vi "Dresden R2R Sputter 03.02.2018 IY24.vi"() -> ()   [LabVIEW 2009] (continued)
          tunnel: w9769 -> [w9795 w9871 w9895 w9919 w9956 w9990 w10014]
          tunnel: w9772 -> [w9794 w9870 w9894 w9918 w9955 w9989 w10013]
          frame #0 {
            n6486 = stacked-sequence {
              tunnel: [_ _ _ w9837 _] -> w9797
              tunnel: [_ _ _ w9828 _] -> w9796
              tunnel: w9795 -> [_ w9800 _ _ _]
              tunnel: w9794 -> [_ w9799 _ _ _]
              frame #0 {
                n6487 = Wait (ms)(milliseconds to wait=i32? 50) -> ()  [unwired: 1 out]
              }
              frame #1 {
                n6488 = Concatenate Strings("#003A:" ("string"), "\n", "\n") -> (w9818)
                n6489 = VISA Write(VISA resource name=w9800, write buffer=w9818, error in (no error)=w9799) -> (VISA resource name out=w9816, error out=w9815)  [unwired: 1 out]
                n6490 = stacked-sequence {
                  tunnel: [w9823] -> w9814
                  tunnel: w9816 -> [w9823]
                  tunnel: [w9822] -> w9813
                  tunnel: w9815 -> [w9822]
                  frame #0 {
                    n6491 = Wait (ms)(milliseconds to wait=i32? 50) -> ()  [unwired: 1 out]
                  }
                }
                n6492 = property class="Instr"(reference=w9814, error in=w9813) -> (reference out=w9810, error out=w9812, "Serial Settings:Number of Bytes at Serial Port"=w9811)
                n6493 = VISA Read(VISA resource name=w9810, byte count=w9811, error in (no error)=w9812) -> (VISA resource name out=w9802, read buffer=w9804, error out=w9801)  [unwired: 1 out]
                "read buffer 6" <- w9804
                n6494 = Match Pattern(string=w9804, regular expression="#003A:") -> (after substring=w9808)  [unwired: 1 in, 3 out]
                n6495 = String Subset(string=w9808, offset (0)=data[5B], length (rest)=i32? 3 ("length (rest)")) -> (substring=w9805)
                n6496 = Decimal String To Number(string=w9805) -> (number=→"Pc_bv3_position")  [unwired: 2 in, 1 out]
              }
              frame #2 {
                n6497 = Wait (ms)(milliseconds to wait=i32? 50) -> ()  [unwired: 1 out]
              }
              frame #3 {
                n6498 = Concatenate Strings("#003P:" ("string"), "\n", "\n") -> (w9851)
                n6499 = VISA Write(VISA resource name=w9836, write buffer=w9851, error in (no error)=w9835) -> (VISA resource name out=w9849, error out=w9848)  [unwired: 1 out]
                n6500 = stacked-sequence {
                  tunnel: [w9857] -> w9847
                  tunnel: w9849 -> [w9857]
                  tunnel: [w9856] -> w9846
                  tunnel: w9848 -> [w9856]
                  frame #0 {
                    n6501 = Wait (ms)(milliseconds to wait=i32? 50) -> ()  [unwired: 1 out]
                  }
                }
                n6502 = property class="Instr"(reference=w9847, error in=w9846) -> (reference out=w9843, error out=w9845, "Serial Settings:Number of Bytes at Serial Port"=w9844)
                n6503 = VISA Read(VISA resource name=w9843, byte count=w9844, error in (no error)=w9845) -> (VISA resource name out=w9837, read buffer=w9838, error out=w9828)  [unwired: 1 out]
                "read buffer 7" <- w9838
                n6504 = Match Pattern(string=w9838, regular expression="#003P:") -> (after substring=w9829)  [unwired: 1 in, 3 out]
                n6505 = String Subset(string=w9829, offset (0)=i32? 2, length (rest)=i32? 4 ("length (rest)")) -> (substring=w9839)
                n6506 = String Subset(string=w9829, offset (0)=data[5B], length (rest)=i32? 1 ("length (rest)")) -> (substring=w9827)
                n6507 = Equal?(x=w9827, y="-" ("substring")) -> (x = y?=w9825)
                n6508 = Decimal String To Number(string=w9839) -> (number=w9834)  [unwired: 2 in, 1 out]
                n6509 = case shown="True" w9825 {
                  frame #0 {
                  }
                  frame #1 {
                    w9854 = data[5B] ("Pressure_ch3")
                    n6510 = local write "Pressure_ch3"(w9854) -> ()
                    n6511 = local write "Pressure ch3_gui"(w9854) -> ()
                    n6512 = local write "Pressure ch3_gui2"(w9854) -> ()
                  }
                }
                n6513 = Divide(x=w9834, y=i32? 100) -> (x/y=→"Pressure_ch3" →"Pressure ch3_gui" →"Pressure ch3_gui2")
              }
              frame #4 {
                n6514 = Wait (ms)(milliseconds to wait=i32? 50) -> ()  [unwired: 1 out]
              }
            }
          }
          frame #1 {
            n6515 = Concatenate Strings("#003O:" ("string"), "\n", "\n") -> (w9874)
            n6516 = VISA Write(VISA resource name=w9871, write buffer=w9874, error in (no error)=w9870) -> (VISA resource name out=w9860, error out=w9862)  [unwired: 1 out]
            n6517 = stacked-sequence {
              tunnel: [w9882] -> w9869
              tunnel: w9860 -> [w9882]
              tunnel: [w9881] -> w9868
              tunnel: w9862 -> [w9881]
              frame #0 {
                n6518 = Wait (ms)(milliseconds to wait=i32? 50) -> ()  [unwired: 1 out]
              }
            }
            n6519 = property class="Instr"(reference=w9869, error in=w9868) -> (reference out=w9865, error out=w9867, "Serial Settings:Number of Bytes at Serial Port"=w9866)
            n6520 = local write "Pc_bv3_auto_open"(i16? 0 ("Pc_bv3_auto_open")) -> ()
            n6521 = VISA Read(VISA resource name=w9865, byte count=w9866, error in (no error)=w9867) -> (VISA resource name out=w9864, error out=w9863)  [unwired: 2 out]
            n6522 = stacked-sequence {
              tunnel: [w9879] -> w9859
              tunnel: w9864 -> [w9879]
              tunnel: [w9878] -> w9861
              tunnel: w9863 -> [w9878]
              frame #0 {
                n6523 = Wait (ms)(milliseconds to wait=i32? 50) -> ()  [unwired: 1 out]
              }
            }
          }
          frame #2 {
            n6524 = Concatenate Strings("#003C:" ("string"), "\n", "\n") -> (w9898)
            n6525 = VISA Write(VISA resource name=w9895, write buffer=w9898, error in (no error)=w9894) -> (VISA resource name out=w9886, error out=w9885)  [unwired: 1 out]
            n6526 = stacked-sequence {
              tunnel: [w9906] -> w9893
              tunnel: w9886 -> [w9906]
              tunnel: [w9905] -> w9892
              tunnel: w9885 -> [w9905]
              frame #0 {
                n6527 = Wait (ms)(milliseconds to wait=i32? 50) -> ()  [unwired: 1 out]
              }
            }
            n6528 = local write "Pc_bv3_auto_close"(i16? 0 ("Pc_bv3_auto_close")) -> ()
            n6529 = property class="Instr"(reference=w9893, error in=w9892) -> (reference out=w9889, error out=w9891, "Serial Settings:Number of Bytes at Serial Port"=w9890)
            n6530 = VISA Read(VISA resource name=w9889, byte count=w9890, error in (no error)=w9891) -> (VISA resource name out=w9888, error out=w9887)  [unwired: 2 out]
            n6531 = stacked-sequence {
              tunnel: [w9903] -> w9884
              tunnel: w9888 -> [w9903]
              tunnel: [w9902] -> w9883
              tunnel: w9887 -> [w9902]
              frame #0 {
                n6532 = Wait (ms)(milliseconds to wait=i32? 50) -> ()  [unwired: 1 out]
              }
            }
          }
          frame #3 {
            n6533 = In Range and Coerce(upper limit=dbl? 100.0, x="Set_position_value 3", lower limit=data[9B]) -> (coerced(x)=w9924)  [unwired: 1 out]
            n6534 = Multiply(x=w9924, y=dbl? 1000.0) -> (x*y=w9928)
            n6535 = Number To Decimal String(number=w9928) -> (decimal integer string=w9930)  [unwired: 1 out]
            n6536 = Concatenate Strings("000000" ("string"), w9930) -> (w9932)
            n6537 = String Length(string=w9932) -> (length=w9933)
            n6538 = Subtract(x=w9933, y=i32? 6) -> (x-y=w9935)
            n6539 = String Subset(string=w9932, offset (0)=w9935) -> (substring=w9925)  [unwired: 1 out]
            n6540 = Concatenate Strings("#003R:" ("string"), w9925, "\n", "\n") -> (w9937)
            n6541 = VISA Write(VISA resource name=w9919, write buffer=w9937, error in (no error)=w9918) -> (VISA resource name out=w9912, error out=w9910)  [unwired: 1 out]
            n6542 = stacked-sequence {
              tunnel: [w9942] -> w9911
              tunnel: w9912 -> [w9942]
              tunnel: w9910 -> [w9941]
              tunnel: [w9941] -> w9909
              frame #0 {
                n6543 = Wait (ms)(milliseconds to wait=i32? 50) -> ()  [unwired: 1 out]
              }
            }
            n6544 = property class="Instr"(reference=w9911, error in=w9909) -> (reference out=w9915, error out=w9917, "Serial Settings:Number of Bytes at Serial Port"=w9916)
            n6545 = VISA Read(VISA resource name=w9915, byte count=w9916, error in (no error)=w9917) -> (VISA resource name out=w9914, error out=w9913)  [unwired: 2 out]
            n6546 = local write "Pc_bv3_auto_set position"(i16? 0 ("Pc_bv3_auto_set position")) -> ()
            n6547 = stacked-sequence {
              tunnel: [w9940] -> w9908
              tunnel: w9914 -> [w9940]
              tunnel: [w9939] -> w9907
              tunnel: w9913 -> [w9939]
              frame #0 {
                n6548 = Wait (ms)(milliseconds to wait=i32? 50) -> ()  [unwired: 1 out]
              }
            }
          }
          frame #4 {
            n6549 = Multiply(x="Set_pressure_value 3", y=dbl? 10000.0) -> (x*y=w9962)
            n6550 = Number To Decimal String(number=w9962) -> (decimal integer string=w9964)  [unwired: 1 out]
            n6551 = Concatenate Strings("00000000" ("string"), w9964) -> (w9966)
            n6552 = String Length(string=w9966) -> (length=w9967)
            n6553 = Subtract(x=w9967, y=i32? 8) -> (x-y=w9969)
            n6554 = String Subset(string=w9966, offset (0)=w9969) -> (substring=w9959)  [unwired: 1 out]
            n6555 = Concatenate Strings("#003S:" ("string"), w9959, "\n", "\n") -> (w9971)
            n6556 = VISA Write(VISA resource name=w9956, write buffer=w9971, error in (no error)=w9955) -> (VISA resource name out=w9948, error out=w9946)  [unwired: 1 out]
            n6557 = stacked-sequence {
              tunnel: [w9976] -> w9949
              tunnel: w9948 -> [w9976]
              tunnel: [w9975] -> w9947
              tunnel: w9946 -> [w9975]
              frame #0 {
                n6558 = Wait (ms)(milliseconds to wait=i32? 50) -> ()  [unwired: 1 out]
              }
            }
            n6559 = property class="Instr"(reference=w9949, error in=w9947) -> (reference out=w9952, error out=w9954, "Serial Settings:Number of Bytes at Serial Port"=w9953)
            n6560 = local write "Pc_bv3_auto_set_pressure"(i16? 0 ("Pc_bv3_auto_set_pressure")) -> ()
            n6561 = VISA Read(VISA resource name=w9952, byte count=w9953, error in (no error)=w9954) -> (VISA resource name out=w9951, error out=w9950)  [unwired: 2 out]
            n6562 = stacked-sequence {
              tunnel: [w9974] -> w9945
              tunnel: w9951 -> [w9974]
              tunnel: [w9973] -> w9944
              tunnel: w9950 -> [w9973]
              frame #0 {
                n6563 = Wait (ms)(milliseconds to wait=i32? 50) -> ()  [unwired: 1 out]
              }
            }
          }
          frame #5 {
            n6564 = Concatenate Strings("#003Z:" ("string"), "\n", "\n") -> (w9993)
            n6565 = VISA Write(VISA resource name=w9990, write buffer=w9993, error in (no error)=w9989) -> (VISA resource name out=w9982, error out=w9980)  [unwired: 1 out]
            n6566 = stacked-sequence {
              tunnel: [w10000] -> w9983
              tunnel: w9982 -> [w10000]
              tunnel: [w9999] -> w9981
              tunnel: w9980 -> [w9999]
              frame #0 {
                n6567 = Wait (ms)(milliseconds to wait=i32? 50) -> ()  [unwired: 1 out]
              }
            }
            n6568 = local write "Pc_bv3_auto_baratron_set_zero"(i16? 0 ("Pc_bv3_auto_baratron_set_zero")) -> ()
            n6569 = property class="Instr"(reference=w9983, error in=w9981) -> (reference out=w9986, error out=w9988, "Serial Settings:Number of Bytes at Serial Port"=w9987)
            n6570 = VISA Read(VISA resource name=w9986, byte count=w9987, error in (no error)=w9988) -> (VISA resource name out=w9985, error out=w9984)  [unwired: 2 out]
            n6571 = stacked-sequence {
              tunnel: [w9998] -> w9979
              tunnel: w9985 -> [w9998]
              tunnel: [w9997] -> w9978
              tunnel: w9984 -> [w9997]
              frame #0 {
                n6572 = Wait (ms)(milliseconds to wait=i32? 50) -> ()  [unwired: 1 out]
              }
            }
          }
          frame #6 {
            n6573 = Concatenate Strings("#003s:" ("string"), "string", "\n", "\n") -> (w10019)
            n6574 = VISA Write(VISA resource name=w10014, write buffer=w10019, error in (no error)=w10013) -> (VISA resource name out=w10006, error out=w10004)  [unwired: 1 out]
            n6575 = stacked-sequence {
              tunnel: [w10024] -> w10007
              tunnel: w10006 -> [w10024]
              tunnel: [w10023] -> w10005
              tunnel: w10004 -> [w10023]
              frame #0 {
                n6576 = Wait (ms)(milliseconds to wait=i32? 50) -> ()  [unwired: 1 out]
              }
            }
            n6577 = property class="Instr"(reference=w10007, error in=w10005) -> (reference out=w10010, error out=w10012, "Serial Settings:Number of Bytes at Serial Port"=w10011)
            n6578 = VISA Read(VISA resource name=w10010, byte count=w10011, error in (no error)=w10012) -> (VISA resource name out=w10009, error out=w10008)  [unwired: 2 out]
            n6579 = stacked-sequence {
              tunnel: [w10022] -> w10003
              tunnel: w10009 -> [w10022]
              tunnel: [w10021] -> w10002
              tunnel: w10008 -> [w10021]
              frame #0 {
                n6580 = Wait (ms)(milliseconds to wait=i32? 50) -> ()  [unwired: 1 out]
              }
            }
          }
        }
      }
      frame #3 {
        n6581 = Compound Arithmetic op=OR("Pc_bv4_open", "Pc_bv_open_ch4_gui", "Pc_bv4_auto_open", "Pc_bv4_open 2") -> (w10032)
        n6582 = Or(x="Pc_bv4_set position", y="Pc_bv4_auto_set position") -> (x .or. y?=w10043)
        n6583 = Or(x="Pc_bv4_set_pressure", y="Pc_bv4_auto_set_pressure") -> (x .or. y?=w10042)
        n6584 = Or(x="Pc_bv4_auto_baratron_set_zero", y="Baratron_set_zero") -> (x .or. y?=w10041)
        n6585 = Compound Arithmetic op=OR("Pc_bv4_close", "Pc_bv_close_ch4_gui", "Pc_bv4_auto_close", "Pc_bv4_close 2") -> (w10033)
        n6586 = Build Array(i16? 0, w10032, w10033, w10043, w10042, w10041) -> (w10040)
        n6587 = Boolean Array To Number(Boolean array=w10040) -> (number=w10052)
        n6588 = Mantissa & Exponent(0:w10052) -> (2:w10051)  [unwired: 1 out]
        n6589 = case shown="3" w10051 {
          tunnel: [w10056 w10119 w10143 w10166 w10205 w10238] -> w10031
          tunnel: [w10055 w10118 w10142 w10167 w10204 w10237] -> w10030
          tunnel: w10029 -> [w10054 w10130 w10154 w10178 w10216 w10249]
          tunnel: w10028 -> [w10053 w10129 w10153 w10177 w10215 w10248]
          frame #0 {
            n6590 = stacked-sequence {
              tunnel: [_ _ _ w10096 _] -> w10056
              tunnel: [_ _ _ w10095 _] -> w10055
              tunnel: w10054 -> [_ w10059 _ _ _]
              tunnel: w10053 -> [_ w10058 _ _ _]
              frame #0 {
                n6591 = Wait (ms)(milliseconds to wait=i32? 50) -> ()  [unwired: 1 out]
              }
              frame #1 {
                n6592 = Concatenate Strings("#004A:" ("string"), "\n", "\n") -> (w10077)
                n6593 = VISA Write(VISA resource name=w10059, write buffer=w10077, error in (no error)=w10058) -> (VISA resource name out=w10075, error out=w10074)  [unwired: 1 out]
                n6594 = stacked-sequence {
                  tunnel: [w10082] -> w10073
                  tunnel: w10075 -> [w10082]
                  tunnel: [w10081] -> w10072
                  tunnel: w10074 -> [w10081]
                  frame #0 {
                    n6595 = Wait (ms)(milliseconds to wait=i32? 50) -> ()  [unwired: 1 out]
                  }
                }
                n6596 = property class="Instr"(reference=w10073, error in=w10072) -> (reference out=w10069, error out=w10071, "Serial Settings:Number of Bytes at Serial Port"=w10070)
                n6597 = VISA Read(VISA resource name=w10069, byte count=w10070, error in (no error)=w10071) -> (VISA resource name out=w10061, read buffer=w10063, error out=w10060)  [unwired: 1 out]
                "read buffer 8" <- w10063
                n6598 = Match Pattern(string=w10063, regular expression="#004A:") -> (after substring=w10067)  [unwired: 1 in, 3 out]
                n6599 = String Subset(string=w10067, offset (0)=data[5B], length (rest)=i32? 3 ("length (rest)")) -> (substring=w10064)
                n6600 = Decimal String To Number(string=w10064) -> (number=→"Pc_bv4_position")  [unwired: 2 in, 1 out]
              }
              frame #2 {
                n6601 = Wait (ms)(milliseconds to wait=i32? 50) -> ()  [unwired: 1 out]
              }
              frame #3 {
                n6602 = Concatenate Strings("#004P:" ("string"), "\n", "\n") -> (w10110)
                n6603 = VISA Write(VISA resource name=w10094, write buffer=w10110, error in (no error)=w10090) -> (VISA resource name out=w10108, error out=w10107)  [unwired: 1 out]
                n6604 = stacked-sequence {
                  tunnel: [w10116] -> w10106
                  tunnel: w10108 -> [w10116]
                  tunnel: [w10115] -> w10105
                  tunnel: w10107 -> [w10115]
                  frame #0 {
                    n6605 = Wait (ms)(milliseconds to wait=i32? 50) -> ()  [unwired: 1 out]
                  }
                }
                n6606 = property class="Instr"(reference=w10106, error in=w10105) -> (reference out=w10102, error out=w10104, "Serial Settings:Number of Bytes at Serial Port"=w10103)
                n6607 = VISA Read(VISA resource name=w10102, byte count=w10103, error in (no error)=w10104) -> (VISA resource name out=w10096, read buffer=w10097, error out=w10095)  [unwired: 1 out]
                "read buffer 9" <- w10097
                n6608 = Match Pattern(string=w10097, regular expression="#004P:") -> (after substring=w10084)  [unwired: 1 in, 3 out]
                n6609 = String Subset(string=w10084, offset (0)=data[5B], length (rest)=i32? 1 ("length (rest)")) -> (substring=w10087)
                n6610 = String Subset(string=w10084, offset (0)=i32? 2, length (rest)=i32? 4 ("length (rest)")) -> (substring=w10098)
                n6611 = Equal?(x=w10087, y="-") -> (x = y?=w10085)
                n6612 = Decimal String To Number(string=w10098) -> (number=w10093)  [unwired: 2 in, 1 out]
                n6613 = case shown="True" w10085 {
                  frame #0 {
                  }
                  frame #1 {
                    w10113 = data[5B] ("Pressure 4")
                    n6614 = local write "Pressure 4"(w10113) -> ()
                    n6615 = local write "Pressurech4_gui"(w10113) -> ()
                    n6616 = local write "Pressurech4_gui 2"(w10113) -> ()
                  }
                }
                n6617 = Divide(x=w10093, y=i32? 100) -> (x/y=→"Pressure 4" →"Pressurech4_gui" →"Pressurech4_gui 2")
              }
              frame #4 {
                n6618 = Wait (ms)(milliseconds to wait=i32? 50) -> ()  [unwired: 1 out]
              }
            }
          }
          frame #1 {
            n6619 = Concatenate Strings("#004O:" ("string"), "\n", "\n") -> (w10133)
            n6620 = VISA Write(VISA resource name=w10130, write buffer=w10133, error in (no error)=w10129) -> (VISA resource name out=w10122, error out=w10120)  [unwired: 1 out]
            n6621 = stacked-sequence {
              tunnel: [w10140] -> w10123
              tunnel: w10122 -> [w10140]
              tunnel: [w10139] -> w10121
              tunnel: w10120 -> [w10139]
              frame #0 {
                n6622 = Wait (ms)(milliseconds to wait=i32? 50) -> ()  [unwired: 1 out]
              }
            }
            n6623 = local write "Pc_bv4_auto_open"(i16? 0 ("Pc_bv4_auto_open")) -> ()
            n6624 = property class="Instr"(reference=w10123, error in=w10121) -> (reference out=w10126, error out=w10128, "Serial Settings:Number of Bytes at Serial Port"=w10127)
            n6625 = VISA Read(VISA resource name=w10126, byte count=w10127, error in (no error)=w10128) -> (VISA resource name out=w10125, error out=w10124)  [unwired: 2 out]
            n6626 = stacked-sequence {
              tunnel: [w10138] -> w10119
              tunnel: w10125 -> [w10138]
              tunnel: [w10137] -> w10118
              tunnel: w10124 -> [w10137]
              frame #0 {
                n6627 = Wait (ms)(milliseconds to wait=i32? 50) -> ()  [unwired: 1 out]
              }
            }
          }
          frame #2 {
            n6628 = Concatenate Strings("#004C:" ("string"), "\n", "\n") -> (w10157)
            n6629 = VISA Write(VISA resource name=w10154, write buffer=w10157, error in (no error)=w10153) -> (VISA resource name out=w10145, error out=w10144)  [unwired: 1 out]
            n6630 = local write "Pc_bv4_auto_close"(i16? 0 ("Pc_bv4_auto_close")) -> ()
            n6631 = stacked-sequence {
              tunnel: [w10164] -> w10147
              tunnel: w10145 -> [w10164]
              tunnel: [w10163] -> w10146
              tunnel: w10144 -> [w10163]
              frame #0 {
                n6632 = Wait (ms)(milliseconds to wait=i32? 50) -> ()  [unwired: 1 out]
              }
            }
            n6633 = property class="Instr"(reference=w10147, error in=w10146) -> (reference out=w10150, error out=w10152, "Serial Settings:Number of Bytes at Serial Port"=w10151)
            n6634 = VISA Read(VISA resource name=w10150, byte count=w10151, error in (no error)=w10152) -> (VISA resource name out=w10149, error out=w10148)  [unwired: 2 out]
            n6635 = stacked-sequence {
              tunnel: [w10162] -> w10143
              tunnel: w10149 -> [w10162]
              tunnel: [w10161] -> w10142
              tunnel: w10148 -> [w10161]
              frame #0 {
                n6636 = Wait (ms)(milliseconds to wait=i32? 50) -> ()  [unwired: 1 out]
              }
            }
          }
          frame #3 {
            n6637 = In Range and Coerce(upper limit=dbl? 100.0, x="Set_position_value 4", lower limit=data[9B]) -> (coerced(x)=w10181)  [unwired: 1 out]
            n6638 = Multiply(x=w10181, y=dbl? 1000.0) -> (x*y=w10188)
            n6639 = Number To Decimal String(number=w10188) -> (decimal integer string=w10189)  [unwired: 1 out]
            n6640 = Concatenate Strings("000000" ("string"), w10189) -> (w10191)
            n6641 = String Length(string=w10191) -> (length=w10192)
            n6642 = Subtract(x=w10192, y=i32? 6) -> (x-y=w10194)
            n6643 = String Subset(string=w10191, offset (0)=w10194) -> (substring=w10185)  [unwired: 1 out]
            n6644 = Concatenate Strings("#004R:" ("string"), w10185, "\n", "\n") -> (w10196)
            n6645 = VISA Write(VISA resource name=w10178, write buffer=w10196, error in (no error)=w10177) -> (VISA resource name out=w10169, error out=w10168)  [unwired: 1 out]
            n6646 = stacked-sequence {
              tunnel: [w10201] -> w10171
              tunnel: w10169 -> [w10201]
              tunnel: [w10200] -> w10170
              tunnel: w10168 -> [w10200]
              frame #0 {
                n6647 = Wait (ms)(milliseconds to wait=i32? 50) -> ()  [unwired: 1 out]
              }
            }
            n6648 = property class="Instr"(reference=w10171, error in=w10170) -> (reference out=w10174, error out=w10176, "Serial Settings:Number of Bytes at Serial Port"=w10175)
            n6649 = local write "Pc_bv4_auto_set position"(i16? 0 ("Pc_bv4_auto_set position")) -> ()
            n6650 = VISA Read(VISA resource name=w10174, byte count=w10175, error in (no error)=w10176) -> (VISA resource name out=w10173, error out=w10172)  [unwired: 2 out]
            n6651 = stacked-sequence {
              tunnel: [w10199] -> w10166
              tunnel: w10173 -> [w10199]
              tunnel: [w10198] -> w10167
              tunnel: w10172 -> [w10198]
              frame #0 {
                n6652 = Wait (ms)(milliseconds to wait=i32? 50) -> ()  [unwired: 1 out]
              }
            }
          }
          frame #4 {
            n6653 = Multiply(x="Set_pressure_value 4", y=dbl? 10000.0) -> (x*y=w10221)
            n6654 = Number To Decimal String(number=w10221) -> (decimal integer string=w10223)  [unwired: 1 out]
            n6655 = Concatenate Strings("00000000" ("string"), w10223) -> (w10225)
            n6656 = String Length(string=w10225) -> (length=w10226)
            n6657 = Subtract(x=w10226, y=i32? 8) -> (x-y=w10228)
            n6658 = String Subset(string=w10225, offset (0)=w10228) -> (substring=w10218)  [unwired: 1 out]
            n6659 = Concatenate Strings("#004S:" ("string"), w10218, "\n", "\n") -> (w10230)
            n6660 = VISA Write(VISA resource name=w10216, write buffer=w10230, error in (no error)=w10215) -> (VISA resource name out=w10207, error out=w10206)  [unwired: 1 out]
            n6661 = stacked-sequence {
              tunnel: [w10235] -> w10209
              tunnel: w10207 -> [w10235]
              tunnel: [w10234] -> w10208
              tunnel: w10206 -> [w10234]
              frame #0 {
                n6662 = Wait (ms)(milliseconds to wait=i32? 50) -> ()  [unwired: 1 out]
              }
            }
            n6663 = property class="Instr"(reference=w10209, error in=w10208) -> (reference out=w10212, error out=w10214, "Serial Settings:Number of Bytes at Serial Port"=w10213)
            n6664 = local write "Pc_bv4_auto_set_pressure"(i16? 0 ("Pc_bv4_auto_set_pressure")) -> ()
            n6665 = VISA Read(VISA resource name=w10212, byte count=w10213, error in (no error)=w10214) -> (VISA resource name out=w10211, error out=w10210)  [unwired: 2 out]
            n6666 = stacked-sequence {
              tunnel: [w10233] -> w10205
              tunnel: w10211 -> [w10233]
              tunnel: [w10232] -> w10204
              tunnel: w10210 -> [w10232]
              frame #0 {
                n6667 = Wait (ms)(milliseconds to wait=i32? 50) -> ()  [unwired: 1 out]
              }
            }
          }
          frame #5 {
            n6668 = Concatenate Strings("#004Z:" ("string"), "\n", "\n") -> (w10252)
            n6669 = VISA Write(VISA resource name=w10249, write buffer=w10252, error in (no error)=w10248) -> (VISA resource name out=w10239, error out=w10240)  [unwired: 1 out]
            n6670 = stacked-sequence {
              tunnel: [w10259] -> w10242
              tunnel: w10239 -> [w10259]
              tunnel: [w10258] -> w10241
              tunnel: w10240 -> [w10258]
              frame #0 {
                n6671 = Wait (ms)(milliseconds to wait=i32? 50) -> ()  [unwired: 1 out]
              }
            }
            n6672 = local write "Pc_bv4_auto_baratron_set_zero"(i16? 0 ("Pc_bv4_auto_baratron_set_zero")) -> ()
            n6673 = property class="Instr"(reference=w10242, error in=w10241) -> (reference out=w10245, error out=w10247, "Serial Settings:Number of Bytes at Serial Port"=w10246)
            n6674 = VISA Read(VISA resource name=w10245, byte count=w10246, error in (no error)=w10247) -> (VISA resource name out=w10244, error out=w10243)  [unwired: 2 out]
            n6675 = stacked-sequence {
              tunnel: [w10257] -> w10238
              tunnel: w10244 -> [w10257]
              tunnel: [w10256] -> w10237
              tunnel: w10243 -> [w10256]
              frame #0 {
                n6676 = Wait (ms)(milliseconds to wait=i32? 50) -> ()  [unwired: 1 out]
              }
            }
          }
        }
      }
    }
    n6677 = Wait Until Next ms Multiple(millisecond multiple=i32? 300) -> ()  [unwired: 1 out]
  }
  n6678 = while {
    tunnel: w833 -> [w10265]
    tunnel: w832 -> [w10264]
    tunnel: [w10263] -> w811
    tunnel: [w10262] -> w810
    i -> [w10261]
    stop <- i16? 0 stop-if-true
    n6679 = Wait Until Next ms Multiple(millisecond multiple=i32? 300) -> ()  [unwired: 1 out]
    n6680 = stacked-sequence {
      tunnel: w10265 -> [w10320]
      tunnel: w10264 -> [w10298]
      tunnel: [w10297] -> w10263
      tunnel: [w10296] -> w10262
      tunnel: w10261 -> [w10304]
      frame #0 {
        n6681 = Compound Arithmetic op=OR("Dc_off", "Dc_auto_off", "Dc_off 2") -> (w10291)
        n6682 = Compound Arithmetic op=OR("Dc_host_auto", "DC_host", "DC_host 2") -> (w10268)
        n6683 = Compound Arithmetic op=OR("Dc_set", "Dc_set 2", "Dc_auto_set") -> (w10287)
        n6684 = Compound Arithmetic op=OR("Dc_auto_set_zero", "Dc_set_zero", "Dc_set_zero 2") -> (w10288)
        n6685 = Boolean To (0,1)(Boolean=w10291) -> (0, 1=w10300)
        n6686 = Boolean To (0,1)(Boolean=w10268) -> (0, 1=w10299)
        n6687 = Compound Arithmetic op=OR("Dc_auto_off_ramp_up", "DC_ramp_up", "DC_ramp_up 2") -> (w10289)
        n6688 = Compound Arithmetic op=OR("Dc_auto_ramp_down", "DC_ramp_down", "DC_ramp_down 2") -> (w10290)
        n6689 = Compound Arithmetic op=OR("Dc_on", "Dc_auto_on", "Dc_on 2") -> (w10292)
        n6690 = Boolean To (0,1)(Boolean=w10288) -> (0, 1=w10324)
        n6691 = Boolean To (0,1)(Boolean=w10287) -> (0, 1=w10328)
        n6692 = Multiply(x=w10299, y=i16? 1) -> (x*y=w10321)
        n6693 = Boolean To (0,1)(Boolean="DC_auto_voltage_mode") -> (0, 1=w10308)
        n6694 = Boolean To (0,1)(Boolean=w10289) -> (0, 1=w10318)
        n6695 = Boolean To (0,1)(Boolean=w10290) -> (0, 1=w10315)
        n6696 = Boolean To (0,1)(Boolean="DC_auto_power_mode") -> (0, 1=w10312)
        n6697 = Multiply(x=w10300, y=i16? 3) -> (x*y=w10329)
        n6698 = Multiply(x=w10324, y=i16? 5) -> (x*y=w10323)
        n6699 = Multiply(x=w10328, y=i16? 4) -> (x*y=w10326)
        n6700 = Multiply(x=w10308, y=i16? 9) -> (x*y=w10307)
        n6701 = Multiply(x=w10318, y=i16? 6) -> (x*y=w10314)
        n6702 = Multiply(x=w10315, y=i16? 7) -> (x*y=w10313)
        n6703 = Multiply(x=w10312, y=i16? 8) -> (x*y=w10310)
        n6704 = Boolean To (0,1)(Boolean=w10292) -> (0, 1=w10333)
        n6705 = Multiply(x=w10333, y=i16? 2) -> (x*y=w10331)
        n6706 = Compound Arithmetic op=ADD(w10321, w10331, w10329, w10326, w10323, w10314, w10313, w10310, w10307) -> (w10319)
        n6707 = Quotient & Remainder(x=w10304, y=i32? 5) -> (x-y*floor(x/y)=w10302)  [unwired: 1 out]
        n6708 = Equal To 0?(x=w10302) -> (x = 0?=w10301)
        n6709 = case shown="0, Default" w10319 {
          tunnel: w10320 -> [w10338 w10421 w10428 w10436 w10450 w10474 w10501 w10528 w10551 w10558]
          tunnel: w10298 -> [w10337 w10420 w10427 w10435 w10449 w10473 w10500 w10527 w10550 w10557]
          tunnel: [w10335 w10419 w10425 w10434 w10445 w10472 w10499 w10526 w10549 w10556] -> w10297
          tunnel: [w10334 w10418 w10424 w10433 w10444 w10471 w10498 w10525 w10548 w10555] -> w10296
          tunnel: w10301 -> [w10336 _ _ _ _ _ _ _ _ _]
          frame #0 {
            n6710 = case shown="True" w10336 {
              tunnel: w10338 -> [w10342 w10388]
              tunnel: w10337 -> [w10341 w10387]
              tunnel: [w10340 w10384] -> w10335
              tunnel: [w10339 w10385] -> w10334
              frame #0 {
                n6711 = VISA Write(VISA resource name=w10342, write buffer=bytes[3], error in (no error)=w10341) -> (VISA resource name out=w10365, error out=w10366)  [unwired: 1 out]
                n6712 = stacked-sequence {
                  tunnel: [w10382] -> w10363
                  tunnel: w10365 -> [w10382]
                  tunnel: [w10381] -> w10362
                  tunnel: w10366 -> [w10381]
                  frame #0 {
                    n6713 = Wait Until Next ms Multiple(millisecond multiple=i32? 40) -> ()  [unwired: 1 out]
                  }
                }
                n6714 = property class="Instr"(reference=w10363, error in=w10362) -> (reference out=w10357, error out=w10359, "Serial Settings:Number of Bytes at Serial Port"=w10358)
                n6715 = VISA Read(VISA resource name=w10357, byte count=w10358, error in (no error)=w10359) -> (VISA resource name out=w10340, read buffer=w10372, error out=w10339)  [unwired: 1 out]
                "read buffer" <- w10372
                n6716 = String Length(string=w10372) -> (length=w10371)
                n6717 = Match Pattern(string=w10372, regular expression="¥") -> (after substring=w10344)  [unwired: 4 out]
                n6718 = Equal To 0?(x=w10371) -> (x = 0?=w10370)
                n6719 = String Subset(string=w10344, length (rest)=i32? 2 ("length (rest)")) -> (substring=w10354)  [unwired: 1 out]
                n6720 = String To Byte Array(string=w10354) -> (unsigned byte array=w10360)
                n6721 = Index Array(array=w10360, index=i32? 1) -> (element=w10349)
                n6722 = Index Array(array=w10360, index=data[5B]) -> (element=w10347)
                n6723 = To Unsigned Long Integer(number=w10349) -> (unsigned 32bit integer=w10351)
                n6724 = To Unsigned Long Integer(number=w10347) -> (unsigned 32bit integer=w10346)
                n6725 = Multiply(x=i32? 256, y=w10351) -> (x*y=w10348)
                n6726 = String Length(string=w10344) -> (length=w10361)
                n6727 = Not Equal To 0?(x=w10361) -> (x != 0?=w10343)
                n6728 = Add(x=w10348, y=w10346) -> (x+y=w10345)
                n6729 = feedback #158() -> (w10368)  [unwired: 1 in]
                n6730 = case shown="True" w10370 {
                  tunnel: [T/1 i16? 0] -> w10369
                  tunnel: w10368 -> [_ w10379]
                  tunnel: [i16? 0 w10376] -> w10367
                  frame #0 {
                  }
                  frame #1 {
                    n6731 = call "Elapsed Time130"(2:w10379) -> (16:w10377)  [unwired: 11 in, 7 out]
                    n6732 = Greater?(x=w10377, y=dbl? 6.0) -> (0:w10376)
                  }
                }
                n6733 = case shown="True" w10343 {
                  tunnel: w10345 -> [_ w10383]
                  frame #0 {
                  }
                  frame #1 {
                    "Actual DC Power" <- w10383
                    "Actual DC Power : 2" <- w10383
                  }
                }
                n6734 = local write "Dcps_fail"(w10367) -> ()
              }
              frame #1 {
                n6735 = VISA Write(VISA resource name=w10388, write buffer=bytes[3], error in (no error)=w10387) -> (VISA resource name out=w10411, error out=w10412)  [unwired: 1 out]
                n6736 = stacked-sequence {
                  tunnel: [w10415] -> w10403
                  tunnel: w10411 -> [w10415]
                  tunnel: [w10414] -> w10404
                  tunnel: w10412 -> [w10414]
                  frame #0 {
                    n6737 = Wait Until Next ms Multiple(millisecond multiple=i32? 40) -> ()  [unwired: 1 out]
                  }
                }
                n6738 = property class="Instr"(reference=w10403, error in=w10404) -> (reference out=w10390, error out=w10391, "Serial Settings:Number of Bytes at Serial Port"=w10389)
                n6739 = VISA Read(VISA resource name=w10390, byte count=w10389, error in (no error)=w10391) -> (VISA resource name out=w10384, read buffer=w10410, error out=w10385)  [unwired: 1 out]
                n6740 = Match Pattern(string=w10410, regular expression="¦") -> (after substring=w10409)  [unwired: 4 out]
                n6741 = String Length(string=w10409) -> (length=w10405)
                n6742 = String Subset(string=w10409, length (rest)=i32? 2 ("length (rest)")) -> (substring=w10394)  [unwired: 1 out]
                n6743 = Not Equal To 0?(x=w10405) -> (x != 0?=w10408)
                n6744 = String To Byte Array(string=w10394) -> (unsigned byte array=w10406)
                n6745 = Index Array(array=w10406, index=i32? 1) -> (element=w10398)
                n6746 = Index Array(array=w10406, index=data[5B]) -> (element=w10401)
                n6747 = To Unsigned Long Integer(number=w10398) -> (unsigned 32bit integer=w10399)
                n6748 = To Unsigned Long Integer(number=w10401) -> (unsigned 32bit integer=w10402)
                n6749 = Multiply(x=i32? 256, y=w10399) -> (x*y=w10400)
                n6750 = Add(x=w10400, y=w10402) -> (x+y=w10407)
                n6751 = case shown="True" w10408 {
                  tunnel: w10407 -> [_ w10413]
                  frame #0 {
                  }
                  frame #1 {
                    # "Volt"
                    "Actual DC Volt :" <- w10413
                    "Actual DC Volt2" <- w10413
                  }
                }
              }
            }
          }
          frame #1 {
            # "Host kontrol"
            n6752 = local write "Dc_host_auto"(i16? 0 ("Dc_host_auto")) -> ()
            n6753 = VISA Write(VISA resource name=w10421, write buffer=bytes[4], error in (no error)=w10420) -> (VISA resource name out=w10419, error out=w10418)  [unwired: 1 out]
          }
          frame #2 {
            n6754 = local read "Dcps_fail"() -> (w10426)
            n6755 = case shown="False" w10426 {
              frame #0 {
                "Dcps_is_on" <- T/1 ("Dcps_is_on")
              }
              frame #1 {
              }
            }
            n6756 = local write "Dc_auto_on"(i16? 0 ("Dc_auto_on")) -> ()
            n6757 = VISA Write(VISA resource name=w10428, write buffer=bytes[3], error in (no error)=w10427) -> (VISA resource name out=w10425, error out=w10424)  [unwired: 1 out]
          }
          frame #3 {
            w10431 = data[9B] ("Dc_set_pow")
            n6758 = local write "Set DC Power       : 2"(w10431) -> ()
            n6759 = local write "Set DC Power       :"(w10431) -> ()
            n6760 = flat-sequence {
              frame #0 {
                n6761 = Wait (ms)(milliseconds to wait=i32? 100) -> ()  [unwired: 1 out]
              }
              frame #1 {
                n6762 = local write "Dcps_is_on"(i16? 0 ("DC_auto_off")) -> ()
              }
            }
            n6763 = local write "Dc_auto_off"(i16? 0 ("Dc_auto_off")) -> ()
            n6764 = VISA Write(VISA resource name=w10436, write buffer=bytes[3], error in (no error)=w10435) -> (VISA resource name out=w10434, error out=w10433)  [unwired: 1 out]
          }
          frame #4 {
            w10446 = dbl? 2000.0 ("y")
            n6765 = Or(x="Set DC Power       : 2", y="Set DC Power       :") -> (x .or. y?=w10441)
            n6766 = Less Or Equal?(x=w10441, y=w10446) -> (x <= y?=w10447)
            n6767 = Select(t=w10441, s=w10447, f=w10446) -> (s? t:f=w10448)
            n6768 = Quotient & Remainder(x=w10448, y=dbl? 256.0) -> (x-y*floor(x/y)=w10465, floor(x/y)=w10464)
            n6769 = Build Array(w10465) -> (w10457)
            n6770 = Build Array(w10464) -> (w10459)
            n6771 = Byte Array To String(unsigned byte array=w10457) -> (string=w10458)
            n6772 = Byte Array To String(unsigned byte array=w10459) -> (string=w10460)
            n6773 = Concatenate Strings(bytes[2], w10458, w10460) -> (w10455)
            n6774 = String To Byte Array(string=w10455) -> (unsigned byte array=w10451)
            n6775 = for {
              tunnel: w10451 -> [w10468] mode=indexing
              shift-right: [w10466] -> w10453
              shift-left: data[5B] -> [w10467]
              n6776 = Exclusive Or(1:w10467, 2:w10468) -> (0:w10466)
            }
            n6777 = local write "Dc_auto_set"(i16? 0 ("Dc_auto_set")) -> ()
            n6778 = Build Array(w10453) -> (w10463)
            n6779 = Byte Array To String(unsigned byte array=w10463) -> (string=w10454)
            n6780 = Concatenate Strings(w10455, w10454) -> (w10461)
            n6781 = VISA Write(VISA resource name=w10450, write buffer=w10461, error in (no error)=w10449) -> (VISA resource name out=w10445, error out=w10444)  [unwired: 1 out]
          }
          frame #5 {
            w10469 = data[9B] ("Dc_set_pow")
            n6782 = local write "Set DC Power       : 2"(w10469) -> ()
            n6783 = local write "Set DC Power       :"(w10469) -> ()
            n6784 = Quotient & Remainder(x=data[9B], y=dbl? 256.0) -> (x-y*floor(x/y)=w10489, floor(x/y)=w10488)
            n6785 = Build Array(w10489) -> (w10481)
            n6786 = Build Array(w10488) -> (w10483)
            n6787 = Byte Array To String(unsigned byte array=w10481) -> (string=w10482)
            n6788 = Byte Array To String(unsigned byte array=w10483) -> (string=w10484)
            n6789 = Concatenate Strings(bytes[2], w10482, w10484) -> (w10479)
            n6790 = String To Byte Array(string=w10479) -> (unsigned byte array=w10475)
            n6791 = for {
              tunnel: w10475 -> [w10493] mode=indexing
              shift-right: [w10491] -> w10477
              shift-left: data[5B] -> [w10492]
              n6792 = Exclusive Or(1:w10492, 2:w10493) -> (0:w10491)
            }
            n6793 = local write "Dc_auto_set_zero"(i16? 0 ("Dc_auto_set_zero")) -> ()
            n6794 = Build Array(w10477) -> (w10487)
            n6795 = Byte Array To String(unsigned byte array=w10487) -> (string=w10478)
            n6796 = Concatenate Strings(w10479, w10478) -> (w10485)
            n6797 = VISA Write(VISA resource name=w10474, write buffer=w10485, error in (no error)=w10473) -> (VISA resource name out=w10472, error out=w10471)  [unwired: 1 out]
          }
          frame #6 {
            n6798 = Or(x="DC_ramp_up_time :", y="DC_ramp_up_time : 2") -> (x .or. y?=w10495)
            n6799 = Multiply(x=w10495, y=dbl? 10.0) -> (x*y=w10505)
            n6800 = To Unsigned Long Integer(number=w10505) -> (unsigned 32bit integer=w10502)
            n6801 = Quotient & Remainder(x=w10502, y=i32? 256) -> (x-y*floor(x/y)=w10508, floor(x/y)=w10507)
            n6802 = Build Array(w10508, w10507) -> (w10504)
            n6803 = Byte Array To String(unsigned byte array=w10504) -> (string=w10511)
            n6804 = Concatenate Strings(bytes[2], w10511) -> (w10512)
            n6805 = String To Byte Array(string=w10512) -> (unsigned byte array=w10517)
            n6806 = for {
              tunnel: w10517 -> [w10520] mode=indexing
              shift-right: [w10518] -> w10515
              shift-left: data[5B] -> [w10519]
              n6807 = Exclusive Or(1:w10519, 2:w10520) -> (0:w10518)
            }
            n6808 = local write "Dc_auto_off_ramp_up"(i16? 0 ("Dc_auto_off_ramp_up")) -> ()
            n6809 = Build Array(w10515) -> (w10503)
            n6810 = Byte Array To String(unsigned byte array=w10503) -> (string=w10513)
            n6811 = Concatenate Strings(w10512, w10513) -> (w10510)
            n6812 = VISA Write(VISA resource name=w10501, write buffer=w10510, error in (no error)=w10500) -> (VISA resource name out=w10499, error out=w10498)  [unwired: 1 out]
          }
          frame #7 {
            n6813 = Or(x="DC_ramp_down_time: 2", y="DC_ramp_down_time:") -> (x .or. y?=w10522)
            n6814 = Multiply(x=w10522, y=dbl? 10.0) -> (x*y=w10532)
            n6815 = To Unsigned Long Integer(number=w10532) -> (unsigned 32bit integer=w10529)
            n6816 = Quotient & Remainder(x=w10529, y=i32? 256) -> (x-y*floor(x/y)=w10535, floor(x/y)=w10534)
            n6817 = Build Array(w10535, w10534) -> (w10531)
            n6818 = Byte Array To String(unsigned byte array=w10531) -> (string=w10538)
            n6819 = Concatenate Strings("\n ", w10538) -> (w10539)
            n6820 = String To Byte Array(string=w10539) -> (unsigned byte array=w10544)
            n6821 = for {
              tunnel: w10544 -> [w10547] mode=indexing
              shift-right: [w10545] -> w10542
              shift-left: data[5B] -> [w10546]
              n6822 = Exclusive Or(1:w10546, 2:w10547) -> (0:w10545)
            }
            n6823 = local write "Dc_auto_ramp_down"(i16? 0 ("Dc_auto_ramp_down")) -> ()
            n6824 = Build Array(w10542) -> (w10530)
            n6825 = Byte Array To String(unsigned byte array=w10530) -> (string=w10540)
            n6826 = Concatenate Strings(w10539, w10540) -> (w10537)
            n6827 = VISA Write(VISA resource name=w10528, write buffer=w10537, error in (no error)=w10527) -> (VISA resource name out=w10526, error out=w10525)  [unwired: 1 out]
          }
          frame #8 {
            n6828 = flat-sequence {
              frame #0 {
                n6829 = Wait (ms)(milliseconds to wait=i32? 100) -> ()  [unwired: 1 out]
              }
              frame #1 {
                n6830 = local write "DC_auto_power_mode"(i16? 0 ("DC_auto_power_mode")) -> ()
              }
            }
            n6831 = VISA Write(VISA resource name=w10551, write buffer=bytes[4], error in (no error)=w10550) -> (VISA resource name out=w10549, error out=w10548)  [unwired: 1 out]